vi "HFRR ADV v039 new software.vi"() -> ()   [LabVIEW 2025] (continued)
                  frame False {
                    n2630 = local write "acq timer"(w3142) -> ()
                    n2631 = local write "Test Duration Status"(0.0 ("Test Duration Status")) -> ()
                  }
                  frame True {
                    n2632 = local read "Set Hz"() -> (w3156:dbl)
                    n2633 = local write "Elapsed time"(w3149) -> ()
                    n2634 = local read "test time"() -> (w3148:dbl)
                    n2635 = Multiply(x=w3159, y=w3156) -> (x*y=w3158:dbl)
                    n2636 = case shown="False" w3154 {
                      tunnel: w3158 -> [w3160 _]
                      tunnel: [w3160 1.0] -> w3155
                      frame False {
                        n2637 = local write "Cycles elapsed"(w3160) -> ()
                      }
                      frame True {
                      }
                    }
                    n2638 = Greater?(x=w3149, y=w3148) -> (0:w3157:bool)
                    n2639 = Subtract(x=w3148, y=w3149) -> (x-y=w3147:dbl)
                    n2640 = Multiply(x=w3147, y=60.0) -> (x*y=w3146:dbl)
                    n2641 = local write "Time Remaining"(w3146) -> ()
                    n2642 = local write "Remaining Time"(w3146) -> ()
                    n2643 = case shown="True" w3157 {
                      frame False {
                      }
                      frame True {
                        n2644 = stacked-sequence {
                          frame #0 {
                            w3165 = T19."Enabled" ("Disabled")
                            w3164 = FALSE ("TEST FILE NAM,E SAVED")
                            w3166 = "" ("FILE")
                            w3167 = TRUE ("Visible")
                            n2645 = local write "RUN"(FALSE ("OK Button 2")) -> ()
                            n2646 = local write "Heater Button"(FALSE ("Heater Button")) -> ()
                            n2647 = local write "Auto Start Test"(FALSE ("Auto Start Test")) -> ()
                            n2648 = local write "TestCompFlg"(TRUE ("StpFlg")) -> ()
                            n2649 = local read "Humidity ( %RH )"() -> (→"Rh After":dbl)
                            n2650 = property on="STOP 2" class="Bool (strict)"("Disabled"=u8 0) -> ()  [unwired: 2 in, 2 out]
                            n2651 = local read "EVENT LOG"() -> (w3172:string)
                            n2652 = call "Event Log.vi"("Content"="Test Completed", "EVENT LOG"=w3172) -> ("EVENT LOG"=w3171:string)  [unwired: 8 in, 1 out]
                            n2653 = property on="RUN" class="Bool (strict)"("Visible"=w3167) -> ()  [unwired: 2 in, 2 out]
                            n2654 = property on="Auto Start Test" class="Bool (strict)"("Visible"=w3167) -> ()  [unwired: 2 in, 2 out]
                            n2655 = local write "Batch Ref Num :"(w3166) -> ()
                            n2656 = local write "FILE"(w3166) -> ()
                            n2657 = local write "EVENT LOG"(w3171) -> ()
                            n2658 = local write "TEST FILE NAM,E SAVED"(w3164) -> ()
                            n2659 = local write "Fuel Discription :"(w3166) -> ()
                            n2660 = local write "START TEMP"(w3164) -> ()
                            n2661 = local write "Remarks :"(w3166) -> ()
                            n2662 = local write "Main Dashboard Buttons"(T1."Imaging" ("Main Dashboard Buttons")) -> ()
                            n2663 = local write "Main Tab"(T2."Adv Scar" ("Main Tab")) -> ()
                            n2664 = property on="FRICVALZ 2" class="Bool (strict)"("DisabledEnum"=w3165) -> ()  [unwired: 2 in, 2 out]
                            n2665 = property on="FRICVALZ 3" class="Bool (strict)"("DisabledEnum"=w3165) -> ()  [unwired: 2 in, 2 out]
                            n2666 = property on="FRICVALZ 4" class="Bool (strict)"("DisabledEnum"=w3165) -> ()  [unwired: 2 in, 2 out]
                          }
                          frame #1 {
                            n2667 = Wait (ms)(milliseconds to wait=u32 1500) -> ()  [unwired: 1 out]
                          }
                          frame #2 {
                            n2668 = local read "WriteHumidity"() -> (w3180:string[])
                            n2669 = Insert Into Array(array=w3180, new element="R;1" ("new element/subarray")) -> (w3178:string[])  [unwired: 1 in]
                            n2670 = local write "Due Write"("VC;0") -> ()
                            n2671 = local write "WriteHumidity"(w3178) -> ()
                          }
                          frame #3 {
                            n2672 = Wait (ms)(milliseconds to wait=u32 1500) -> ()  [unwired: 1 out]
                          }
                          frame #4 {
                            n2673 = local read "WriteHumidity"() -> (w3185:string[])
                            n2674 = Insert Into Array(array=w3185, new element="R;1" ("new element/subarray")) -> (w3184:string[])  [unwired: 1 in]
                            n2675 = local write "Due Write"("VC;0") -> ()
                            n2676 = local write "WriteHumidity"(w3184) -> ()
                          }
                          frame #5 {
                            n2677 = Wait (ms)(milliseconds to wait=u32 1500) -> ()  [unwired: 1 out]
                          }
                          frame #6 {
                            n2678 = local write "Due Write"("ST;0") -> ()
                          }
                          frame #7 {
                            n2679 = local write "measured_stroke"(0.0 ("measured_stroke")) -> ()
                            n2680 = Wait (ms)(milliseconds to wait=u32 1500) -> ()  [unwired: 1 out]
                          }
                          frame #8 {
                            n2681 = local write "Humidity"(FALSE ("Humidity")) -> ()
                            n2682 = local write "Due Write"("HE;0") -> ()
                          }
                          frame #9 {
                            n2683 = local write "HUMIDITY CLEAR"(TRUE ("HUMIDITY CLEAR")) -> ()
                          }
                        }
                      }
                    }
                    n2684 = Divide(x=w3149, y=w3148) -> (x/y=w3152:dbl)
                    n2685 = Multiply(x=w3152, y=100.0) -> (x*y=w3150:dbl)
                    n2686 = local write "Test Duration Status"(w3150) -> ()
                  }
                }
              }
              frame #2 {
                n2687 = case shown="True" "Heater Button" {
                  tunnel: [0.0 ("output") w3293] -> w3271
                  frame False {
                    w3274 = TRUE ("tmpchk")
                    n2688 = local read "TEMP"() -> (w3275:dbl)
                    n2689 = local write "Reset 4"(w3274) -> ()
                    n2690 = local write "tmpchk"(w3274) -> ()
                    n2691 = local write "Temp ini"(w3275) -> ()
                    n2692 = local write "reinit"(TRUE ("reinit")) -> ()
                    n2693 = local write "manual temp log"(TRUE ("manual temp log")) -> ()
                  }
                  frame True {
                    # "Logic to turn off\nthe heater when \ntemp is not rising.\nTime - 60 sec\nDelta t- 5°c"
                    n2694 = local read "Temp ini"() -> (w3282:dbl)
                    n2695 = local read "Auto Start Test"() -> (w3278:bool)
                    n2696 = Less?(x=w3282, y=53.0) -> (x < y?=w3280:bool)
                    n2697 = case shown="False" w3278 {
                      frame False {
                        n2698 = local read "Set Temp"() -> (w3302:dbl)
                        n2699 = local read "TEMP"() -> (w3301:dbl)
                        n2700 = Subtract(x=w3302, y=w3301) -> (x-y=w3300:dbl)
                        n2701 = Absolute Value(x=w3300) -> (abs(x)=w3299:dbl)
                        n2702 = Less?(x=w3299, y=0.5) -> (x < y?=w3297:bool)
                        n2703 = case shown="True" w3297 {
                          tunnel: "manual temp log" -> [_ w3303]
                          frame False {
                          }
                          frame True {
                            n2704 = case shown="True" w3303 {
                              selector: w3303 -> [_ w3304]
                              frame False {
                              }
                              frame True {
                                # "#Event log"
                                n2705 = Not(x=w3304) -> (.not. x?=w3305:bool)
                                n2706 = local write "manual temp log"(w3305) -> ()
                                n2707 = local read "EVENT LOG"() -> (w3308:string)
                                n2708 = call "Event Log.vi"("Content"="Target Temperature reached", "EVENT LOG"=w3308) -> ("EVENT LOG"=w3307:string)  [unwired: 8 in, 1 out]
                                n2709 = local write "EVENT LOG"(w3307) -> ()
                              }
                            }
                          }
                        }
                      }
                      frame True {
                        n2710 = local write "manual temp log"(TRUE ("manual temp log")) -> ()
                      }
                    }
                    n2711 = And(x="tmpchk", y=w3280) -> (x .and. y?=w3283:bool)
                    n2712 = case shown="True" w3283 {
                      frame False {
                      }
                      frame True {
                        n2713 = call "Elapsed Time8"("Time Target (s)"=300.0, "Reset"="Reset 4") -> ("Time has Elapsed"=w3310:bool)  [unwired: 10 in, 7 out]
                        n2714 = flat-sequence {
                          tunnel: w3310 -> [_]
                          frame #0 {
                            n2715 = local write "Reset 4"(FALSE ("Reset 4")) -> ()
                          }
                        }
                        n2716 = case shown="True" w3310 {
                          frame False {
                          }
                          frame True {
                            n2717 = local read "Temp ini"() -> (w3317:dbl)
                            n2718 = Add(x=w3317, y=5.0) -> (x+y=w3315:dbl)
                            n2719 = local read "TEMP"() -> (w3318:dbl)
                            n2720 = Greater?(x=w3318, y=w3315) -> (0:w3316:bool)
                            n2721 = case shown="False" w3316 {
                              frame False {
                                n2722 = local write "Heater Button"(FALSE ("Heater Button")) -> ()
                              }
                              frame True {
                                n2723 = local write "tmpchk"(FALSE ("tmpchk")) -> ()
                              }
                            }
                          }
                        }
                      }
                    }
                    n2724 = local read "Set Temp"() -> (w3291:dbl)
                    n2725 = local read "TEMP"() -> (w3285:dbl)
                    n2726 = call-poly <vilib>:"PID.vi"("reinitialize? (F)"="reinit", "dt (s)"=-1.0, "process variable"=w3285, "setpoint"=w3291) -> ("output"=w3288:dbl)  [unwired: 6 in, 1 out]
                    n2727 = Subtract(x=w3291, y=w3285) -> (x-y=w3292:dbl)
                    n2728 = Add(x=w3291, y=0.5) -> (x+y=w3289:dbl)
                    n2729 = Greater Or Equal?(x=w3285, y=w3289) -> ()  [unwired: 1 out]
                    n2730 = Select(t=0.0, s=FALSE, f=w3288) -> (s? t:f=w3287:dbl)
                    "PID output" <- w3287
                    n2731 = flat-sequence {
                      tunnel: w3287 -> [w3321]
                      tunnel: [w3321] -> w3293
                      frame #0 {
                        n2732 = local write "reinit"(FALSE ("reinit")) -> ()
                      }
                    }
                    n2733 = Bundle(w3292, "output"=w3287, "TEMP"=w3285) -> ()  [unwired: 1 in, 1 out]
                  }
                }
                "PID-out" <- w3271
              }
              frame #3 {
                n2734 = local read "TEMP"() -> (w3323:dbl)
                n2735 = Greater Or Equal?(x=w3323, y="Set Temp 2") -> (x >= y?=w3328:bool)
                n2736 = case shown="True" w3328 {
                  tunnel: [FALSE TRUE] -> w3326
                  frame False {
                  }
                  frame True {
                  }
                }
                "Status 13" <- w3326
                n2737 = And(x=w3326, y="trip1 8") -> (x .and. y?=w3325:bool)
                n2738 = case shown="True" w3325 {
                  frame False {
                    n2739 = local write "Heater Trip Temp"(TRUE ("Heater Trip Temp")) -> ()
                  }
                  frame True {
                    w3331 = FALSE ("OK Button 2")
                    n2740 = case shown="True" "Heater Trip Temp" {
                      selector: "Heater Trip Temp" -> [_ w3333]
                      frame False {
                      }
                      frame True {
                        n2741 = Not(x=w3333) -> (.not. x?=w3332:bool)
                        n2742 = local read "EVENT LOG"() -> (w3336:string)
                        n2743 = local write "Heater Trip Temp"(w3332) -> ()
                        n2744 = call "Event Log.vi"("Content"="Heater Trip", "EVENT LOG"=w3336) -> ("EVENT LOG"=w3335:string)  [unwired: 8 in, 1 out]
                        n2745 = local write "EVENT LOG"(w3335) -> ()
                      }
                    }
                    n2746 = local write "RUN"(w3331) -> ()
                    n2747 = property on="Auto Start Test" class="Bool (strict)"("Value"=w3331) -> ()  [unwired: 2 in, 2 out]
                    n2748 = local write "Heater Button"(w3331) -> ()
                  }
                }
              }
            }
            n2749 = case shown="False" w3037 {
              frame False {
                n2750 = disable-structure shown="Disabled" {
                  frame Disabled {
                    n2751 = stacked-sequence {
                      frame #0 {
                        n2752 = local write "RUN"(FALSE ("OK Button 2")) -> ()
                      }
                      frame #1 {
                      }
                    }
                  }
                  frame Enabled {
                  }
                }
              }
              frame True {
              }
            }
          }
        }
        n2753 = case shown="True" w2934 {
          frame False {
            n2754 = local read "Rt 3"() -> (w3002:bool)
            n2755 = case shown="True" w3002 {
              frame False {
              }
              frame True {
                n2756 = local write "Rt 3"(FALSE ("Rt 3")) -> ()
              }
            }
            "Rt" <- TRUE ("Rt")
            "Rt 2" <- FALSE ("Rt")
          }
          frame True {
            n2757 = local read "Rt"() -> (w3008:bool)
            n2758 = local write "Rt 2"(TRUE ("Rt 2")) -> ()
            n2759 = case shown="True" w3008 {
              frame False {
              }
              frame True {
                n2760 = local write "Rt"(FALSE ("Rt")) -> ()
              }
            }
            "Rt 3" <- TRUE ("Rt 3")
          }
        }
        n2761 = local read "Reset Graph"() -> (w2930:bool)
        n2762 = case shown="True" w2930 {
          selector: w2930 -> [_ w2947]
          frame False {
          }
          frame True {
            w2961 = 0.0 ("X Scale.Range:Maximum")
            n2763 = Not(x=w2947) -> (.not. x?=w2946:bool)
            n2764 = local write "Reset Graph"(w2946) -> ()
            n2765 = property on="Electrical Contact Resistance ( % )" class="WFChart (strict)"("XScale.Maximum"=600.0 ("X Scale.Range:Maximum"), "XScale.Minimum"=0.0 ("X Scale.Range:Minimum"), "YScale.Maximum"=100.0 ("Y Scale.Range:Maximum"), "YScale.Minimum"=0.0 ("Y Scale.Range:Minimum")) -> ()  [unwired: 2 in, 2 out]
            n2766 = property on="Frictional Force ( N )" class="WFChart (strict)"("XScale.Maximum"=600.0 ("X Scale.Range:Maximum"), "XScale.Minimum"=0.0 ("X Scale.Range:Minimum"), "YScale.Maximum"=100.0 ("Y Scale.Range:Maximum"), "YScale.Minimum"=0.0 ("Y Scale.Range:Minimum")) -> ()  [unwired: 2 in, 2 out]
            n2767 = property on="Temperature ( Deg C )" class="WFChart (strict)"("XScale.Maximum"=600.0 ("X Scale.Range:Maximum"), "XScale.Minimum"=0.0 ("X Scale.Range:Minimum"), "YScale.Maximum"=100.0 ("Y Scale.Range:Maximum"), "YScale.Minimum"=0.0 ("Y Scale.Range:Minimum")) -> ()  [unwired: 2 in, 2 out]
            n2768 = property on="Coefficient of Friction" class="WFChart (strict)"("XScale.Maximum"=600.0 ("X Scale.Range:Maximum"), "XScale.Minimum"=0.0 ("X Scale.Range:Minimum"), "YScale.Maximum"=100.0 ("Y Scale.Range:Maximum"), "YScale.Minimum"=0.0 ("Y Scale.Range:Minimum")) -> ()  [unwired: 2 in, 2 out]
            n2769 = property on="Stroke ( mm )" class="WFChart (strict)"("XScale.Maximum"=600.0 ("X Scale.Range:Maximum"), "XScale.Minimum"=0.0 ("X Scale.Range:Minimum"), "YScale.Maximum"=100.0 ("Y Scale.Range:Maximum"), "YScale.Minimum"=0.0 ("Y Scale.Range:Minimum")) -> ()  [unwired: 2 in, 2 out]
            n2770 = property on="Electrical Contact Resistance ( % )" class="WFChart (strict)"("XScale.Minimum"=0.0 ("X Scale.Range:Minimum"), "XScale.Maximum"=600.0 ("X Scale.Range:Maximum"), "YScale.Minimum"=0.0 ("Y Scale.Range:Minimum"), "YScale.Maximum"=100.0 ("Y Scale.Range:Maximum")) -> ()  [unwired: 2 in, 2 out]
            n2771 = property on="Temperature ( Deg C )" class="WFChart (strict)"("XScale.Minimum"=0.0 ("X Scale.Range:Minimum"), "XScale.Maximum"=600.0 ("X Scale.Range:Maximum"), "YScale.Minimum"=0.0 ("Y Scale.Range:Minimum"), "YScale.Maximum"=100.0 ("Y Scale.Range:Maximum")) -> ()  [unwired: 2 in, 2 out]
            n2772 = property on="Coefficient of Friction" class="WFChart (strict)"("XScale.Minimum"=0.0 ("X Scale.Range:Minimum"), "XScale.Maximum"=600.0 ("X Scale.Range:Maximum"), "YScale.Maximum"=1.0 ("X Scale.Range:Minimum"), "YScale.Minimum"=0.0 ("X Scale.Range:Minimum")) -> ()  [unwired: 2 in, 2 out]
            n2773 = property on="Frictional Force ( N )" class="WFChart (strict)"("XScale.Maximum"=600.0 ("X Scale.Range:Maximum"), "XScale.Minimum"=w2961, "YScale.Maximum"=10.0 ("Y Scale.Range:Maximum"), "YScale.Minimum"=w2961) -> ()  [unwired: 2 in, 2 out]
            n2774 = property on="Stroke ( mm )" class="WFChart (strict)"("XScale.Maximum"=600.0 ("X Scale.Range:Maximum"), "XScale.Minimum"=0.0 ("X Scale.Range:Minimum"), "YScale.Maximum"=100.0 ("Y Scale.Range:Maximum"), "YScale.Minimum"=0.0 ("Y Scale.Range:Minimum")) -> ()  [unwired: 2 in, 2 out]
            n2775 = property on="Humidity ( %RH ) 2" class="WFChart (strict)"("XScale.Maximum"=600.0 ("X Scale.Range:Maximum"), "XScale.Minimum"=0.0 ("X Scale.Range:Minimum"), "YScale.Maximum"=100.0 ("Y Scale.Range:Maximum"), "YScale.Minimum"=0.0 ("Y Scale.Range:Minimum")) -> ()  [unwired: 2 in, 2 out]
          }
        }
      }
      frame "Compare Files" {
        # "Elapsed time\ncof\nstroke\nAir temp\nTemp\nHumidity"
        n2776 = case shown="True" "RST CP 3" {
          frame False {
          }
          frame True {
            n2777 = property on="Air Temp ( °C ) vs Humidity ( % RH )" class="XYGraph (strict)"("X Scale.Range:Minimum"=18.0, "X Scale.Range:Maximum"=28.0 ("X Scale.Range:Minimum"), "Y Scale.Range:Minimum"=30.0 ("X Scale.Range:Minimum"), "Y Scale.Range:Maximum"=70.0 ("X Scale.Range:Minimum")) -> ()  [unwired: 2 in, 2 out]
          }
        }
        n2778 = case shown="True" "RST CP 2" {
          frame False {
          }
          frame True {
            n2779 = property on="XY Graph 13" class="XYGraph (strict)"("Y Scale.Display Format:Precision"=u8 0 ("Y Scale.Format & Precision:Precision")) -> ()  [unwired: 2 in, 2 out]
            n2780 = property on="XY Graph 13" class="XYGraph (strict)"("X Scale.Range:Minimum"=0.0, "X Scale.Range:Maximum"=75.0, "Y Scale.Range:Minimum"=0.0, "Y Scale.Range:Maximum"=100.0) -> ()  [unwired: 2 in, 2 out]
          }
        }
        n2781 = case shown="True" "RSTV1 2" {
          frame False {
          }
          frame True {
            n2782 = property on="Humidity ( %RH )" class="XYGraph (strict)"("Y Scale.Display Format:Precision"=u8 0 ("Y Scale.Format & Precision:Precision")) -> ()  [unwired: 2 in, 2 out]
            n2783 = property on="Humidity ( %RH )" class="XYGraph (strict)"("X Scale.Range:Minimum"=0.0, "X Scale.Range:Maximum"=75.0, "Y Scale.Range:Minimum"=48.0, "Y Scale.Range:Maximum"=58.0) -> ()  [unwired: 2 in, 2 out]
          }
        }
        n2784 = case shown="True" "RST CP" {
          frame False {
          }
          frame True {
            n2785 = property on="Sample Temperature ( °C )" class="XYGraph (strict)"("Y Scale.Display Format:Precision"=u8 2 ("Y Scale.Format & Precision:Precision")) -> ()  [unwired: 2 in, 2 out]
            n2786 = property on="Sample Temperature ( °C )" class="XYGraph (strict)"("X Scale.Range:Minimum"=0.0, "X Scale.Range:Maximum"=75.0, "Y Scale.Range:Minimum"=58.0, "Y Scale.Range:Maximum"=62.0) -> ()  [unwired: 2 in, 2 out]
          }
        }
        n2787 = case shown="True" "RSTV1 3" {
          frame False {
          }
          frame True {
            n2788 = property on="Air Temperature  ( °C )" class="XYGraph (strict)"("Y Scale.Display Format:Precision"=u8 2 ("Y Scale.Format & Precision:Precision")) -> ()  [unwired: 2 in, 2 out]
            n2789 = property on="Air Temperature  ( °C )" class="XYGraph (strict)"("X Scale.Range:Minimum"=0.0 ("Y Scale.Range:Minimum"), "X Scale.Range:Maximum"=75.0 ("Y Scale.Range:Maximum"), "Y Scale.Range:Minimum"=20.0 ("X Scale.Range:Minimum"), "Y Scale.Range:Maximum"=26.0 ("X Scale.Range:Maximum")) -> ()  [unwired: 2 in, 2 out]
          }
        }
        n2790 = case shown="True" "rstv2" {
          frame False {
          }
          frame True {
            n2791 = property on="Coefficient Of Friction" class="XYGraph (strict)"("Y Scale.Display Format:Precision"=u8 3 ("Y Scale.Format & Precision:Precision")) -> ()  [unwired: 2 in, 2 out]
            n2792 = property on="Coefficient Of Friction" class="XYGraph (strict)"("X Scale.Range:Minimum"=0.0 ("Y Scale.Range:Maximum"), "X Scale.Range:Maximum"=75.0, "Y Scale.Range:Minimum"=0.0, "Y Scale.Range:Maximum"=1.0 ("X Scale.Range:Minimum")) -> ()  [unwired: 2 in, 2 out]
          }
        }
        n2793 = case shown="True" "RSTV1 4" {
          frame False {
          }
          frame True {
            n2794 = property on="Stroke ( mm )" class="XYGraph (strict)"("Y Scale.Display Format:Precision"=u8 2 ("Y Scale.Format & Precision:Precision")) -> ()  [unwired: 2 in, 2 out]
            n2795 = property on="Stroke ( mm )" class="XYGraph (strict)"("X Scale.Range:Minimum"=0.0 ("Y Scale.Range:Maximum"), "X Scale.Range:Maximum"=75.0 ("X Scale.Range:Minimum"), "Y Scale.Range:Minimum"=0.98, "Y Scale.Range:Maximum"=1.02) -> ()  [unwired: 2 in, 2 out]
          }
        }
        n2796 = case shown="True" "OPEN 1" {
          frame False {
          }
          frame True {
            (unwired) 0  # existing file
            w3612 = "Choose a datalog file to open"  # prompt
            n2797 = local write "OPEN 1"(FALSE ("OPEN 1")) -> ()
            n2798 = String To Path(string="C:\\LAB-IQ\\Data\\") -> (path=w3597:path)
            n2799 = File Dialog(6:"*.dgf" ("pattern"), 7:w3612, 11:w3597) -> (0:w3595:errorcluster, 3:w3603:path)  [unwired: 4 in, 2 out]
            n2800 = Unbundle(w3595) -> ()  [unwired: 3 out]
            n2801 = Strip Path(path=w3603) -> (name=w3602:string)  [unwired: 1 out]
            n2802 = Path To String(path=w3603) -> (string=w3598:string)
            "string1" <- w3598
            n2803 = Match Pattern(string=w3602, regular expression=".dgf") -> (before substring=→"String Control":string)  [unwired: 1 in, 3 out]
            n2804 = Match Pattern(string=w3598, regular expression=".dgf" ("substring (\"\")")) -> (before substring=w3608:string)  [unwired: 1 in, 3 out]
            n2805 = Concatenate Strings(w3608, ".duf" ("Substring")) -> (w3604:string)
            n2806 = String To Path(string=w3604) -> (path=w3609:path)
            n2807 = call <vilib>:"Read Characters From File.vi"("file path (dialog if empty)"=w3609, "start of read offset (chars.:0)"=60 ("start of read offset (chars.: 0)")) -> ("character string"=→"String Control 2":string)  [unwired: 4 in, 3 out]
          }
        }
        n2808 = case shown="True" "OPEN 2" {
          frame False {
          }
          frame True {
            (unwired) 0  # existing file
            w3630 = "Choose a datalog file to open"  # prompt
            n2809 = local write "OPEN 2"(FALSE ("OPEN 1")) -> ()
            n2810 = String To Path(string="C:\\LAB-IQ\\Data\\") -> (path=w3615:path)
            n2811 = File Dialog(6:"*.dgf" ("pattern"), 7:w3630, 11:w3615) -> (0:w3613:errorcluster, 3:w3621:path)  [unwired: 4 in, 2 out]
            n2812 = Unbundle(w3613) -> ()  [unwired: 3 out]
            n2813 = Strip Path(path=w3621) -> (name=w3619:string)  [unwired: 1 out]
            n2814 = Path To String(path=w3621) -> (string=w3616:string)
            "string1 2" <- w3616
            n2815 = Match Pattern(string=w3619, regular expression=".dgf") -> (before substring=→"String Control 3":string)  [unwired: 1 in, 3 out]
            n2816 = Match Pattern(string=w3616, regular expression=".dgf" ("substring (\"\")")) -> (before substring=w3627:string)  [unwired: 1 in, 3 out]
            n2817 = Concatenate Strings(w3627, ".duf" ("Substring")) -> (w3624:string)
            n2818 = String To Path(string=w3624) -> (path=w3622:path)
            n2819 = call <vilib>:"Read Characters From File.vi"("file path (dialog if empty)"=w3622, "start of read offset (chars.:0)"=60 ("start of read offset (chars.: 0)")) -> ("character string"=→"String Control 4":string)  [unwired: 4 in, 3 out]
          }
        }
        n2820 = case shown="True" "OPEN 3" {
          frame False {
          }
          frame True {
            (unwired) 0  # existing file
            w3648 = "Choose a datalog file to open"  # prompt
            n2821 = local write "OPEN 3"(FALSE ("OPEN 1")) -> ()
            n2822 = String To Path(string="C:\\LAB-IQ\\Data\\") -> (path=w3633:path)
            n2823 = File Dialog(6:"*.dgf" ("pattern"), 7:w3648, 11:w3633) -> (0:w3631:errorcluster, 3:w3639:path)  [unwired: 4 in, 2 out]
            n2824 = Unbundle(w3631) -> ()  [unwired: 3 out]
            n2825 = Strip Path(path=w3639) -> (name=w3637:string)  [unwired: 1 out]
            n2826 = Path To String(path=w3639) -> (string=w3634:string)
            "string1 3" <- w3634
            n2827 = Match Pattern(string=w3637, regular expression=".dgf") -> (before substring=→"String Control 5":string)  [unwired: 1 in, 3 out]
            n2828 = Match Pattern(string=w3634, regular expression=".dgf" ("substring (\"\")")) -> (before substring=w3644:string)  [unwired: 1 in, 3 out]
            n2829 = Concatenate Strings(w3644, ".duf" ("Substring")) -> (w3641:string)
            n2830 = String To Path(string=w3641) -> (path=w3645:path)
            n2831 = call <vilib>:"Read Characters From File.vi"("file path (dialog if empty)"=w3645, "start of read offset (chars.:0)"=60 ("start of read offset (chars.: 0)")) -> ("character string"=→"String Control 6":string)  [unwired: 4 in, 3 out]
          }
        }
        n2832 = case shown="True" "OPEN 4" {
          frame False {
          }
          frame True {
            (unwired) 0  # existing file
            w3666 = "Choose a datalog file to open"  # prompt
            n2833 = local write "OPEN 4"(FALSE ("OPEN 1")) -> ()
            n2834 = String To Path(string="C:\\LAB-IQ\\Data\\") -> (path=w3651:path)
            n2835 = File Dialog(6:"*.dgf" ("pattern"), 7:w3666, 11:w3651) -> (0:w3649:errorcluster, 3:w3657:path)  [unwired: 4 in, 2 out]
            n2836 = Unbundle(w3649) -> ()  [unwired: 3 out]
            n2837 = Strip Path(path=w3657) -> (name=w3655:string)  [unwired: 1 out]
            n2838 = Path To String(path=w3657) -> (string=w3652:string)
            "string1 4" <- w3652
            n2839 = Match Pattern(string=w3655, regular expression=".dgf") -> (before substring=→"String Control 7":string)  [unwired: 1 in, 3 out]
            n2840 = Match Pattern(string=w3652, regular expression=".dgf" ("substring (\"\")")) -> (before substring=w3662:string)  [unwired: 1 in, 3 out]
            n2841 = Concatenate Strings(w3662, ".duf" ("Substring")) -> (w3659:string)
            n2842 = String To Path(string=w3659) -> (path=w3663:path)
            n2843 = call <vilib>:"Read Characters From File.vi"("file path (dialog if empty)"=w3663, "start of read offset (chars.:0)"=60 ("start of read offset (chars.: 0)")) -> ("character string"=→"String Control 8":string)  [unwired: 4 in, 3 out]
          }
        }
      }
      frame "About" {
        # "Elapsed time\ncof\nstroke\nmean pos\nTemp\nHumidity"
        n2844 = call <vilib>:"Query Available Printers.vi"() -> ("system configured printers"=w3680:string[])  [unwired: 9 in, 2 out]
        "System Configured Printers 2" <- w3680
        n2845 = local read "OK Button 16"() -> (w3677:bool)
        n2846 = Index Array(array=w3680, index="Select Printer 3") -> (element=w3682:string)
        "Selected Printer" <- w3682
        n2847 = case shown="True" "OK Button 16" {
          frame False {
          }
          frame True {
            n2848 = stacked-sequence {
              frame #0 {
                n2849 = local read "Numeric 16"() -> (w4005:i32)
                n2850 = local write "Numeric 10"(w4005) -> ()
              }
              frame #1 {
                n2851 = local read "String 29"() -> (w4008:string)
                n2852 = String To Path(string=w4008) -> (path=w4007:path)
                n2853 = Open/Create/Replace File "Open File"(file path (use dialog)=w4007) -> (refnum out=w4009:refnum<file>)  [unwired: 5 in, 2 out]
                n2854 = for {
                  N: 16 -> [_]
                  tunnel: w4009 -> [w4016]
                  i -> [w4012]
                  (unwired) TRUE ("line mode (F)")
                  n2855 = Read from Text File "Read File"(file (use dialog)=w4016) -> (text=w4010:string)  [unwired: 3 in, 3 out]
                  n2856 = Match Pattern(string=w4010, regular expression="(") -> (after substring=w4015:string)  [unwired: 1 in, 3 out]
                  n2857 = Match Pattern(string=w4015, regular expression=")") -> (before substring=w4011:string)  [unwired: 1 in, 3 out]
                  n2858 = case shown="1" w4012 {
                    tunnel: w4011 -> [w4017 w4018 _ _ w4019 w4020 w4021 w4023 w4025 w4027 w4029 w4031 w4033 w4035 _]
                    tunnel: w4010 -> [_ _ _ _ _ _ _ _ _ _ _ _ _ _ _]
                    frame 0 {
                      "TITTLE" <- w4017
                    }
                    frame 1 {
                      "Sample ID" <- w4018
                    }
                    frame 2 {
                    }
                    frame 3 {
                    }
                    frame 4 {
                      "Test Date" <- w4019
                    }
                    frame 5 {
                      "Tested by" <- w4020
                    }
                    frame 6 {
                      n2859 = Fract/Exp String To Number(string=w4021) -> (number=→"Humidity before test 2":dbl)  [unwired: 3 in, 1 out]
                    }
                    frame 7 {
                      n2860 = Fract/Exp String To Number(string=w4023) -> (number=→"Temperature before test 2":dbl)  [unwired: 3 in, 1 out]
                    }
                    frame 8 {
                      n2861 = Fract/Exp String To Number(string=w4025) -> (number=→"Humidity after test 2":dbl)  [unwired: 3 in, 1 out]
                    }
                    frame 9 {
                      n2862 = Fract/Exp String To Number(string=w4027) -> (number=→"Temperature after test 2":dbl)  [unwired: 3 in, 1 out]
                    }
                    frame 10 {
                      n2863 = Fract/Exp String To Number(string=w4029) -> (number=→"MWSD 2":dbl)  [unwired: 3 in, 1 out]
                    }
                    frame 11 {
                      n2864 = Fract/Exp String To Number(string=w4031) -> (number=→"AVP 2":dbl)  [unwired: 3 in, 1 out]
                    }
                    frame 12 {
                      n2865 = Fract/Exp String To Number(string=w4033) -> (number=→"HCF 2":dbl)  [unwired: 3 in, 1 out]
                    }
                    frame 13 {
                      n2866 = Fract/Exp String To Number(string=w4035) -> (number=→"WS1.4 2":dbl)  [unwired: 3 in, 1 out]
                    }
                    frame 14, Default {
                    }
                  }
                }
              }
              frame #2 {
              }
            }
            n2867 = local write "OK Button 16"(FALSE ("OK Button 13")) -> ()
          }
        }
        n2868 = disable-structure shown="Disabled" {
          frame Disabled {
            n2869 = case shown="True" "Export" {
              frame False {
              }
              frame True {
                w3688 = "                                      " ("string")
                w3690 = "\r"
                (unwired) i16 6 ("width (-)")
                w3767 = "\r"
                w3699 = "\r"
                n2870 = local write "Export"(FALSE ("Export")) -> ()
                n2871 = local read "String 29"() -> (w3736:string)
                n2872 = local read "String 39"() -> (w3706:string)
                n2873 = local read "String 38"() -> (w3709:string)
                n2874 = local read "String 37"() -> (w3715:string)
                n2875 = local read "String 36"() -> (w3712:string)
                n2876 = local read "String 35"() -> (w3719:string)
                n2877 = local read "String 34"() -> (w3724:string)
                n2878 = Match Pattern(string=w3736, regular expression=".dwm") -> (before substring=w3732:string)  [unwired: 1 in, 3 out]
                "before substring" <- w3732
                n2879 = local read "S 39"() -> (w3720:string)
                n2880 = local read "S 38"() -> (w3727:string)
                n2881 = local read "Temperature before test 2"() -> (w3756:dbl)
                n2882 = local read "Temperature after test 2"() -> (w3761:dbl)
                n2883 = local read "Humidity before test 2"() -> (w3742:dbl)
                n2884 = local read "Humidity after test 2"() -> (w3757:dbl)
                n2885 = local read "MWSD 2"() -> (w3753:dbl)
                n2886 = local read "WS1.4 2"() -> (w3769:dbl)
                n2887 = local read "HCF 2"() -> (w3765:dbl)
                n2888 = local read "AVP 2"() -> (w3754:dbl)
                n2889 = Concatenate Strings("8," ("string"), w3706) -> (w3707:string)
                n2890 = Concatenate Strings("7," ("string"), w3709) -> (w3710:string)
                n2891 = Concatenate Strings("6," ("string"), w3712) -> (w3713:string)
                n2892 = Concatenate Strings("5," ("string"), w3715) -> (w3716:string)
                n2893 = Concatenate Strings("4," ("string"), w3719) -> (w3718:string)
                n2894 = Concatenate Strings("3," ("string"), w3720) -> (w3722:string)
                n2895 = Concatenate Strings("2," ("string"), w3724) -> (w3723:string)
                n2896 = Concatenate Strings("1," ("string"), w3727) -> (w3726:string)
                n2897 = local read "Sample ID"() -> (w3774:string)
                n2898 = case shown="\"xlx\"" "Select File Type" {
                  tunnel: w3732 -> [w3777 w3779 w3781]
                  tunnel: [w3775 w3780 w3782] -> w3731
                  frame "xlx" {
                    n2899 = Concatenate Strings(w3777, ".xls" ("string")) -> (w3775:string)
                  }
                  frame "csv" {
                    n2900 = Concatenate Strings(w3779, ".csv" ("string")) -> (w3780:string)
                  }
                  frame "txt" {
                    n2901 = Concatenate Strings(w3781, ".txt" ("string")) -> (w3782:string)
                  }
                }
                n2902 = local read "Test Date"() -> (w3773:string)
                n2903 = local read "String 45"() -> (w3687:string)
                n2904 = local read "String 31"() -> (w3772:string)
                n2905 = local read "String 32"() -> (w3771:string)
                n2906 = local read "TITTLE"() -> (w3695:string)
                n2907 = Number To Fractional String(number=w3769, precision (6)=i16 2) -> (F-format string=w3770:string)  [unwired: 2 in]
                n2908 = Number To Fractional String(number=w3765, width (-)=i16 6, precision (6)=i16 2) -> (F-format string=w3766:string)  [unwired: 1 in]
                n2909 = Number To Fractional String(number=w3761, width (-)=i16 6, precision (6)=i16 2) -> (F-format string=w3760:string)  [unwired: 1 in]
                n2910 = Number To Fractional String(number=w3754, width (-)=i16 6, precision (6)=i16 2) -> (F-format string=w3752:string)  [unwired: 1 in]
                n2911 = Number To Fractional String(number=w3753, width (-)=i16 6, precision (6)=i16 2) -> (F-format string=w3751:string)  [unwired: 1 in]
                n2912 = Number To Fractional String(number=w3757, width (-)=i16 6, precision (6)=i16 2) -> (F-format string=w3755:string)  [unwired: 1 in]
                n2913 = Number To Fractional String(number=w3756, width (-)=i16 6, precision (6)=i16 2) -> (F-format string=w3762:string)  [unwired: 1 in]
                n2914 = Number To Fractional String(number=w3742, width (-)=i16 6, precision (6)=i16 2) -> (F-format string=w3741:string)  [unwired: 1 in]
                n2915 = local read "s.NO"() -> (w3689:string)
                n2916 = Concatenate Strings("=" ("string"), w3695) -> (w3694:string)
                n2917 = Concatenate Strings("S.No," ("string"), "                                       Parameters" ("string")) -> (w3700:string)
                n2918 = Concatenate Strings(w3767, w3726, w3741, w3767, w3723, w3762, w3767, w3722, w3755, w3767, w3718, w3760, w3767, w3716, w3751, w3767, w3713, w3752, w3767, w3710, w3766, w3767, w3707, w3770) -> (w3729:string)
                n2919 = Concatenate Strings(w3699, "," ("string"), w3687, w3689, w3688, w3771, w3774, w3688, w3772, w3773, w3699) -> (w3697:string)
                n2920 = local read "Tested by"() -> (w3703:string)
                n2921 = local read "String 33"() -> (w3704:string)
                n2922 = Concatenate Strings("," ("string"), "                                                                             " ("string")) -> (w3692:string)
                n2923 = Concatenate Strings(w3694, w3690, w3697, w3690, w3700, w3729, w3690, w3692, w3704, w3703) -> (→"export":string)
                n2924 = String To Path(string=w3731) -> (path=w3738:path)
                n2925 = local read "export"() -> (w3733:string)
                n2926 = call <vilib>:"Write Characters To File.vi"("append to file? (new file:F)"=FALSE, "character string"=w3733, "file path (dialog if empty)"=w3738) -> ()  [unwired: 2 in, 1 out]
              }
            }
          }
          frame Enabled {
          }
        }
        n2927 = case shown="True" "OK Button 17" {
          frame False {
          }
          frame True {
            (unwired) 0  # existing file
            w3991 = "Choose a datalog file to open"  # prompt
            n2928 = local write "OK Button 17"(FALSE ("OK Button 17")) -> ()
            n2929 = local read "String"() -> (w3986:string)
            n2930 = String To Path(string=w3986) -> (path=w3987:path)
            n2931 = File Dialog(6:"*.duf" ("pattern"), 7:w3991, 11:w3987) -> (0:w3978:errorcluster, 3:w3997:path)  [unwired: 4 in, 2 out]
            n2932 = Unbundle(w3978) -> ()  [unwired: 3 out]
            n2933 = Open/Create/Replace File "Open File"(file path (use dialog)=w3997) -> (refnum out=w3989:refnum<file>)  [unwired: 5 in, 2 out]
            n2934 = Strip Path(path=w3997) -> (name=w3995:string)  [unwired: 1 out]
            n2935 = Path To String(path=w3997) -> (string=w3980:string)
            n2936 = local write "String 29"(w3980) -> ()
            n2937 = while {
              tunnel: w3989 -> [w4001]
              i -> [w3998]
              stop <- w3999 continue-if-true
              (unwired) TRUE ("line mode (F)")
              n2938 = Read from Text File "Read File"(file (use dialog)=w4001) -> (text=w4000:string)  [unwired: 3 in, 3 out]
              n2939 = local write "Numeric 16"(w3998) -> ()
              n2940 = String Length(string=w4000) -> (length=w4003:i32)
              n2941 = Greater?(x=w4003, y=1) -> (0:w3999:bool)
            }
            n2942 = Search and Replace String(input string=w3980, search string=".duf", replace string=".dgf" ("replace string (\"\")")) -> (result string=→"String Indicator 4":string)  [unwired: 5 in, 3 out]
            n2943 = Match Pattern(string=w3995, regular expression=".dwm") -> (before substring=w3979:string)  [unwired: 1 in, 3 out]
            "String Indicator" <- w3979
            n2944 = Match Pattern(string=w3980, regular expression=".dwm" ("substring (\"\")")) -> (before substring=w3981:string)  [unwired: 1 in, 3 out]
            "String Indicator 3" <- w3981
            n2945 = local write "TITTLE 2"(w3979) -> ()
            n2946 = String To Path(string=w3981) -> (path=w3988:path)
            "path" <- w3988
            n2947 = call <vilib>:"Read Characters From File.vi"("file path (dialog if empty)"=w3988, "start of read offset (chars.:0)"=60 ("start of read offset (chars.: 0)")) -> ("character string"=→"String Indicator 2":string)  [unwired: 4 in, 3 out]
          }
        }
        n2948 = case shown="True" "Print 2" {
          frame False {
          }
          frame True {
            n2949 = flat-sequence {
              frame #0 {
                n2950 = local read "s.NO"() -> (→"s.NO 2":string)
                n2951 = Wait (ms)(milliseconds to wait=u32 20) -> ()  [unwired: 1 out]
                n2952 = local read "Sample ID  4"() -> (→"Sample ID  7":string)
                n2953 = local read "Sample ID  3"() -> (→"Sample ID  6":string)
                n2954 = local read "Sample ID"() -> (→"Sample ID  2":string)
                n2955 = local read "Tested by"() -> (→"Tested by 2":string)
                n2956 = local read "Test Date"() -> (→"Test Date 2":string)
                n2957 = local read "Humidity after test 3"() -> (→"Humidity after test 4":dbl)
                n2958 = local read "Ref A Test Date :"() -> (→"TITTLE 4":string)
                n2959 = local read "Temperature before test 3"() -> (→"Temperature after test 5":dbl)
                n2960 = local read "Temperature before test 3"() -> (w3799:dbl)
                n2961 = local read "Temperature after test 3"() -> (→"Temperature after test 4":dbl)
                n2962 = local read "Humidity before test 3"() -> (→"Humidity before test 4":dbl)
                n2963 = local write "Temperature before test 3"(w3799) -> ()
                n2964 = local read "image data"() -> (w3790:T16)
                n2965 = String To Path(string="C:\\LAB-IQ\\im\\Temp_resized.jpg") -> (path=w3791:path)
                "path 2" <- w3791
                n2966 = call <vilib>:"Write JPEG File.vi"("image data"=w3790, "path to JPEG file"=w3791) -> ()  [unwired: 8 in, 2 out]
                "Ref A Test Date :" <- "Ref A Test Date :"
                "Ref B Test Date :" <- "Ref B Test Date :"
                "Ref B Scar Value :" <- "Ref B Scar Value :"
                "Ref A Scar Value :" <- "Ref A Scar Value :"
              }
              frame #1 {
                (unwired) HTML_Report_Image_Alignment."MIDDLE" ("alignment (default)")
                w3827 = u16 0 items=["portrait", "landscape"] ("orientation (portrait)")
                (unwired) HTML_Report_Image_Alignment."ABSMIDDLE" ("alignment (default)")
                (unwired) "TESTED BY : "
                (unwired) "TESTED DATE :"
                (unwired) "SAMPLE ID : "
                (unwired) "SAMPLE DESIGN : "
                w3860 = "\r"
                # "add image"
                n2967 = Wait (ms)(milliseconds to wait=u32 20) -> ()  [unwired: 1 out]
                n2968 = local read "Sample ID  2"() -> (w3853:string)
                n2969 = local read "Wear Scar X"() -> (w3825:dbl)
                "Length ( microns ) 2" <- w3825
                n2970 = local read "Wear Scar Y"() -> (w3824:dbl)
                "Wear Scar Y ( microns ) :" <- w3824
                n2971 = local read "Test Date 2"() -> (w3854:string)
                n2972 = local read "Tested by 2"() -> (w3855:string)
                n2973 = local read "String 46"() -> (w3851:string)
                n2974 = local read "String 47"() -> (w3856:string)
                n2975 = local read "String 48"() -> (w3857:string)
                n2976 = local read "String 49"() -> (w3858:string)
                n2977 = local read "String 10"() -> (w3811:string)
                n2978 = local read "s.NO 2"() -> (w3852:string)
                n2979 = Add(x=w3825, y=w3824) -> (x+y=w3823:dbl)
                n2980 = call <vilib>:"New Report.vi"("report type"=enum16{"Standard Report", "HTML"}."HTML") -> ("report out"=w3831:refnum<class "NI_report.lvclass">, "error out"=w3829:errorcluster)  [unwired: 13 in]
                n2981 = Concatenate Strings(w3860, w3851, w3852, w3860, w3857, w3853, w3860, w3856, w3854, w3860, w3858, w3855, w3860) -> (→"test by 2":string)
                n2982 = Concatenate Strings("C:\\LAB-IQ\\Data\\" ("string"), w3811, ".jpg" ("string")) -> ()  [unwired: 1 out]
                n2983 = Divide(x=w3823, y=2.0) -> (x/y=→"Mean Wear ( microns) :":dbl)
                n2984 = call-dynamic "Set Report Orientation.vi"("report in"=w3831, "orientation (portrait)"=w3827, "error in (no error)"=w3829) -> ("report out"=w3830:refnum<class "NI_report.lvclass">, "error out"=w3828:errorcluster)  [unwired: 11 in]
                n2985 = for {
                  N: 5 -> [_]
                  tunnel: w3830 -> [w3881]
                  tunnel: [w3880] -> w3809
                  tunnel: w3828 -> [w3879]
                  tunnel: [w3878] -> w3808
                  n2986 = call-dynamic "Set Report Tab Width.vi"("report in"=w3881, "error in (no error)"=w3879) -> ("report out"=w3880:refnum<class "NI_report.lvclass">, "error out"=w3878:errorcluster)  [unwired: 12 in]
                }
                n2987 = local read "TITTLE"() -> (w3826:string)
                n2988 = call-dynamic "Set Report Header Text.vi"("report in"=w3809, "center header text"=w3826, "error in (no error)"=w3808) -> ("report out"=w3847:refnum<class "NI_report.lvclass">, "error out"=w3846:errorcluster)  [unwired: 11 in]
                n2989 = for {
                  N: 1 -> [_]
                  tunnel: [w3885] -> w3833
                  tunnel: [w3884] -> w3832
                  tunnel: w3847 -> [w3883]
                  tunnel: w3846 -> [w3882]
                  n2990 = call-dynamic "New Report Line.vi"("report in"=w3883, "error in (no error)"=w3882) -> ("report out"=w3885:refnum<class "NI_report.lvclass">, "error out"=w3884:errorcluster)  [unwired: 12 in]
                }
                n2991 = for {
                  N: 2 -> [_]
                  tunnel: [w3877] -> w3839
                  tunnel: [w3876] -> w3838
                  tunnel: w3833 -> [w3875]
                  tunnel: w3832 -> [w3874]
                  n2992 = call-dynamic "New Report Line.vi"("report in"=w3875, "error in (no error)"=w3874) -> ("report out"=w3877:refnum<class "NI_report.lvclass">, "error out"=w3876:errorcluster)  [unwired: 12 in]
                }
                n2993 = for {
                  N: 25 -> [_]
                  tunnel: w3839 -> [w3873]
                  tunnel: w3838 -> [w3871]
                  tunnel: [w3872] -> w3842
                  tunnel: [w3870] -> w3841
                  n2994 = call-dynamic "Set Report Tab Width.vi"("report in"=w3873, "error in (no error)"=w3871) -> ("report out"=w3872:refnum<class "NI_report.lvclass">, "error out"=w3870:errorcluster)  [unwired: 12 in]
                }
                n2995 = control-ref of="Tab Control 9"() -> (w3837:refnum<vi>)
                n2996 = call-dynamic "Append Control Image to Report.vi"("report in"=w3842, "alignment (default)"=HTML_Report_Image_Alignment."ABSMIDDLE", "ctrl reference"=w3837, "error in (no error)"=w3841) -> ("report out"=w3836:refnum<class "NI_report.lvclass">, "error out"=w3835:errorcluster)  [unwired: 8 in, 2 out]
                n2997 = for {
                  N: 3 -> [_]
                  tunnel: [w3869] -> w3820
                  tunnel: [w3868] -> w3819
                  tunnel: w3836 -> [w3867]
                  tunnel: w3835 -> [w3866]
                  n2998 = call-dynamic "New Report Line.vi"("report in"=w3867, "error in (no error)"=w3866) -> ("report out"=w3869:refnum<class "NI_report.lvclass">, "error out"=w3868:errorcluster)  [unwired: 12 in]
                }
                n2999 = for {
                  N: 100 -> [_]
                  tunnel: w3820 -> [w3865]
                  tunnel: w3819 -> [w3863]
                  tunnel: [w3864] -> w3816
                  tunnel: [w3862] -> w3814
                  n3000 = call-dynamic "Set Report Tab Width.vi"("report in"=w3865, "error in (no error)"=w3863) -> ("report out"=w3864:refnum<class "NI_report.lvclass">, "error out"=w3862:errorcluster)  [unwired: 12 in]
                }
                n3001 = String To Path(string="C:\\LAB-IQ\\im\\Temp_resized.jpg") -> (path=w3806:path)
                n3002 = call-poly <vilib>:"Append Image to Report.vi"("report in"=w3816, "path or URL of image"=w3806, "error in (no error)"=w3814) -> ("report out"=w3815:refnum<class "NI_report.lvclass">, "error out"=w3813:errorcluster)  [unwired: 9 in, 2 out]
                n3003 = call-poly <vilib>:"Open HTML Report in Browser.vi"("report in"=w3815, "error in (no error)"=w3813) -> ("report out"=w3850:refnum<class "NI_report.lvclass">, "error out"=w3849:errorcluster)  [unwired: 11 in, 1 out]
                n3004 = call-dynamic "Dispose Report.vi"("report in"=w3850, "error in (no error)"=w3849) -> ()  [unwired: 13 in, 1 out]
              }
              frame #2 {
              }
              frame #3 {
                n3005 = local write "Print 2"(FALSE ("Print")) -> ()
                n3006 = disable-structure shown="Disabled" {
                  frame Disabled {
                    n3007 = local read "String 10"() -> (w3890:string)
                    n3008 = Concatenate Strings("C:\\LAB-IQ-NXT\\Data\\" ("string"), w3890, ".jpg" ("string")) -> (w3888:string)
                    n3009 = String To Path(string=w3888) -> (path=w3887:path)
                    n3010 = Delete(path (use dialog)=w3887) -> ()  [unwired: 4 in, 3 out]
                  }
                  frame Enabled {
                  }
                }
              }
            }
          }
        }
        n3011 = case shown="True" w3677 {
          frame False {
          }
          frame True {
            n3012 = flat-sequence {
              frame #0 {
              }
              frame #1 {
                n3013 = Wait (ms)(milliseconds to wait=u32 100) -> ()  [unwired: 1 out]
              }
              frame #2 {
                n3014 = local write "OK Button 16"(FALSE ("Print 3")) -> ()
              }
            }
          }
        }
        n3015 = case shown="True" "Print" {
          tunnel: w3682 -> [_ w3974]
          frame False {
          }
          frame True {
            (unwired) i16 6 ("width (-)")
            (unwired) "TESTED BY : "
            (unwired) "TESTED DATE :"
            (unwired) "SAMPLE ID : "
            (unwired) "SAMPLE DESIGN : "
            w3932 = "\r"
            w3949 = "\r"
            # "add image"
            n3016 = local read "Sample ID"() -> (w3922:string)
            n3017 = local read "Tested by"() -> (w3925:string)
            n3018 = local read "String 45"() -> (w3892:string)
            n3019 = local read "Test Date"() -> (w3923:string)
            n3020 = local read "String 39"() -> (w3895:string)
            n3021 = local read "String 38"() -> (w3898:string)
            n3022 = local read "String 37"() -> (w3905:string)
            n3023 = local read "String 36"() -> (w3902:string)
            n3024 = local read "String 35"() -> (w3907:string)
            n3025 = local read "String 34"() -> (w3912:string)
            n3026 = local read "String 31"() -> (w3926:string)
            n3027 = local read "String 32"() -> (w3927:string)
            n3028 = local read "String 33"() -> (w3928:string)
            n3029 = local write "Print"(FALSE ("Print FF")) -> ()
            n3030 = local read "S 39"() -> (w3910:string)
            n3031 = local read "S 38"() -> (w3917:string)
            n3032 = local read "Temperature before test 2"() -> (w3948:dbl)
            n3033 = local read "Temperature after test 2"() -> (w3938:dbl)
            n3034 = local read "Humidity before test 2"() -> (w3963:dbl)
            n3035 = local read "Humidity after test 2"() -> (w3947:dbl)
            n3036 = local read "MWSD 2"() -> (w3952:dbl)
            n3037 = local read "WS1.4 2"() -> (w3930:dbl)
            n3038 = Concatenate Strings("8)" ("string"), w3895) -> (w3896:string)
            n3039 = Concatenate Strings("7)" ("string"), w3898) -> (w3899:string)
            n3040 = Concatenate Strings("6)" ("string"), w3902) -> (w3901:string)
            n3041 = Concatenate Strings("5)" ("string"), w3905) -> (w3904:string)
            n3042 = Concatenate Strings("4)" ("string"), w3907) -> (w3908:string)
            n3043 = Concatenate Strings("3)" ("string"), w3910) -> (w3911:string)
            n3044 = Concatenate Strings("2)" ("string"), w3912) -> (w3913:string)
            n3045 = Concatenate Strings("1)" ("string"), w3917) -> (w3916:string)
            n3046 = local read "HCF 2"() -> (w3934:dbl)
            n3047 = local read "AVP 2"() -> (w3951:dbl)
            n3048 = local read "s.NO"() -> (w3893:string)
            n3049 = call <vilib>:"New Report.vi"("report type"=enum16{"Standard Report", "HTML"}."Standard Report") -> ("report out"=w3972:refnum<class "NI_report.lvclass">, "error out"=w3971:errorcluster)  [unwired: 13 in]
            n3050 = local read "TITTLE"() -> (w3924:string)
            n3051 = Concatenate Strings(w3949, w3892, w3893, w3949, w3927, w3922, w3949, w3926, w3923, w3949, w3928, w3925, w3949) -> (w3942:string)
            "test by" <- w3942
            n3052 = Number To Fractional String(number=w3930, precision (6)=i16 2) -> (F-format string=w3929:string)  [unwired: 2 in]
            n3053 = Number To Fractional String(number=w3934, width (-)=i16 6, precision (6)=i16 2) -> (F-format string=w3933:string)  [unwired: 1 in]
            n3054 = Number To Fractional String(number=w3938, width (-)=i16 6, precision (6)=i16 2) -> (F-format string=w3939:string)  [unwired: 1 in]
            n3055 = Number To Fractional String(number=w3951, width (-)=i16 6, precision (6)=i16 2) -> (F-format string=w3953:string)  [unwired: 1 in]
            n3056 = Number To Fractional String(number=w3952, width (-)=i16 6, precision (6)=i16 2) -> (F-format string=w3954:string)  [unwired: 1 in]
            n3057 = Number To Fractional String(number=w3947, width (-)=i16 6, precision (6)=i16 2) -> (F-format string=w3950:string)  [unwired: 1 in]
            n3058 = Number To Fractional String(number=w3948, width (-)=i16 6, precision (6)=i16 2) -> (F-format string=w3937:string)  [unwired: 1 in]
            n3059 = Number To Fractional String(number=w3963, width (-)=i16 6, precision (6)=i16 2) -> (F-format string=w3968:string)  [unwired: 1 in]
            n3060 = call-dynamic "Set Report Header Text.vi"("report in"=w3972, "center header text"=w3924, "error in (no error)"=w3971) -> ("report out"=w3943:refnum<class "NI_report.lvclass">, "error out"=w3944:errorcluster)  [unwired: 11 in]
            n3061 = Concatenate Strings(w3932, w3916, w3968, w3932, w3913, w3937, w3932, w3911, w3950, w3932, w3908, w3939, w3932, w3904, w3954, w3932, w3901, w3953, w3932, w3899, w3933, w3932, w3896, w3929) -> (w3920:string)
            "export 2" <- w3920
            n3062 = call-poly <vilib>:"Append Report Text.vi"("report in"=w3943, "text"=w3942, "error in (no error)"=w3944) -> ("report out"=w3946:refnum<class "NI_report.lvclass">, "error out"=w3945:errorcluster)  [unwired: 9 in, 2 out]
            n3063 = local read "test by"() -> (w3919:string)